vi "FlexMag - 24-03-2023.vi"() -> ()   [LabVIEW 2018] (continued)
              }
              frame True {
                w13696 = FALSE ("CH1_Trns_BP_Left_DO")
                w13698 = FALSE
                w13699 = FALSE
                w13697 = FALSE ("CH1_CC_DO")
                n8105 = local write "Buzzer DO"(TRUE ("Buzzer DO")) -> ()
                n8106 = local write "1-2 tr"(w13699) -> ()
                n8107 = local write "1-3 tr"(w13699) -> ()
                n8108 = local write "1-4 tr"(w13699) -> ()
                n8109 = local write "2-1 tr"(w13699) -> ()
                n8110 = local write "2-3 tr"(w13699) -> ()
                n8111 = local write "2-4 tr"(w13699) -> ()
                n8112 = local write "3-1 tr"(w13699) -> ()
                n8113 = local write "3-2 tr"(w13699) -> ()
                n8114 = local write "3-4 tr"(w13699) -> ()
                n8115 = local write "4-1 tr"(w13699) -> ()
                n8116 = local write "4-2 tr"(w13699) -> ()
                n8117 = local write "4-3 tr"(w13699) -> ()
                n8118 = local write "Casette_Servo_Start/Stop DO"(FALSE ("Casette_Servo_Start/Stop DO")) -> ()
                n8119 = local write "CH3_Trns_BP_Left_DO"(w13696) -> ()
                n8120 = local write "CH3_Trns_BP_Right_DO"(w13696) -> ()
                n8121 = local write "CH3_CC_DO"(w13697) -> ()
                n8122 = local write "ch3 pumpdown alg"(w13697) -> ()
                n8123 = local write "Pump Down CH3"(w13697) -> ()
                n8124 = local write "ch3 shutdown alg"(w13697) -> ()
                n8125 = local write "Shut Down CH3"(w13697) -> ()
                n8126 = local write "ch1-2 transfer"(w13698) -> ()
                n8127 = local write "ch2-3 transfer"(w13698) -> ()
                n8128 = local write "ch3-4 transfer"(w13698) -> ()
                n8129 = local write "ch2-1 transfer"(w13698) -> ()
                n8130 = local write "ch3-2 transfer"(w13698) -> ()
                n8131 = local write "ch4-3 transfer"(w13698) -> ()
              }
            }
            n8132 = case shown="True" w13676 {
              frame False {
              }
              frame True {
                w13692 = TRUE ("Buzzer DO")
                n8133 = local write "Tp3 auto stop"(w13692) -> ()
                n8134 = local write "pcgv3 auto close"(w13692) -> ()
                n8135 = local write "Dc_auto_off"(FALSE ("Dc_auto_off")) -> ()
                n8136 = local write "System Status"("CH3 ABORTED" ("System Status")) -> ()
              }
            }
            n8137 = case shown="True" w13669 {
              frame False {
              }
              frame True {
                n8138 = local write "CH3_PL_VBV_DO"(TRUE) -> ()
                n8139 = local write "CH3_MP_DO"(FALSE ("Buzzer DO")) -> ()
              }
            }
          }
        }
        n8140 = feedback-in #313(w13665) -> ()
      }
    }
  }
  n8141 = VISA Close(VISA resource name=w102, error in (no error)=w101) -> ()  [unwired: 1 out]
  n8142 = VISA Close(VISA resource name=w84, error in (no error)=w85) -> ()  [unwired: 1 out]
  n8143 = VISA Close(VISA resource name=w82, error in (no error)=w83) -> ()  [unwired: 1 out]
  n8144 = VISA Close(VISA resource name=w92, error in (no error)=w91) -> ()  [unwired: 1 out]
  n8145 = while {
    stop <- FALSE stop-if-true
    n8146 = Build Array(FALSE, "ch1-2 transfer", "ch2-3 transfer", "ch3-4 transfer", "ch2-1 transfer", "ch3-2 transfer", "ch4-3 transfer") -> (w13744:bool[])
    n8147 = Boolean Array To Number(Boolean array=w13744) -> (number=w13743:u32)
    n8148 = Wait Until Next ms Multiple(millisecond multiple=u32 300) -> ()  [unwired: 1 out]
    n8149 = Mantissa & Exponent(0:w13743) -> (2:w13742:dbl)  [unwired: 1 out]
    n8150 = case shown="1" w13742 {
      frame 0, Default {
      }
      frame 1 {
        n8151 = local read "ABORT"() -> (w13747:bool)
        n8152 = case shown="False" w13747 {
          frame False {
            n8153 = stacked-sequence {
              frame #0 {
                n8154 = local read "ch1-2 transfer"() -> (w13748:bool)
                n8155 = case shown="True" w13748 {
                  frame False {
                  }
                  frame True {
                    n8156 = local read "present location"() -> (w13751:dbl)
                    n8157 = Wait (ms)(milliseconds to wait=u32 100) -> ()  [unwired: 1 out]
                    n8158 = Equal?(x=w13751, y=1.0) -> (x = y?=w13752:bool)
                    n8159 = case shown="True" w13752 {
                      frame False {
                        n8160 = local write "trns error"(TRUE ("TRNS error")) -> ()
                        n8161 = local write "Warning Message"("Transfer process canceled!\nCassette is not in CH1 " ("Warning Message")) -> ()
                      }
                      frame True {
                        n8162 = local write "System Status"("CH1 to CH2  Transfer in Progress" ("System Status")) -> ()
                      }
                    }
                  }
                }
              }
              frame #1 {
                n8163 = local read "ch1-2 transfer"() -> (w13756:bool)
                n8164 = case shown="True" w13756 {
                  frame False {
                  }
                  frame True {
                    n8165 = stacked-sequence {
                      frame #0 {
                        n8166 = local read "ABORT"() -> (w13757:bool)
                        n8167 = case shown="False" w13757 {
                          frame False {
                            n8168 = local write "trns pre check"(TRUE ("trns pre check")) -> ()
                          }
                          frame True {
                          }
                        }
                      }
                      frame #1 {
                        n8169 = Wait (ms)(milliseconds to wait=u32 1000) -> ()  [unwired: 1 out]
                      }
                      frame #2 {
                        n8170 = while {
                          i -> [w13765]
                          stop <- w13762 stop-if-true
                          # "10 min"
                          n8171 = local read "trns pre check"() -> (w13769:bool)
                          n8172 = local read "ch1-2 transfer"() -> (w13761:bool)
                          n8173 = local read "ABORT"() -> (w13763:bool)
                          n8174 = Greater Or Equal?(x=w13765, y=u32 2000 ("millisecond multiple")) -> (x >= y?=w13764:bool)
                          n8175 = Not(x=w13769) -> (.not. x?=w13768:bool)
                          n8176 = Not(x=w13761) -> (.not. x?=w13760:bool)
                          n8177 = Compound Arithmetic op=OR(w13764, w13768, w13763, w13760) -> (w13762:bool)
                          n8178 = Wait Until Next ms Multiple(millisecond multiple=u32 300) -> ()  [unwired: 1 out]
                        }
                      }
                    }
                  }
                }
              }
              frame #2 {
                n8179 = local read "ch1-2 transfer"() -> (w13770:bool)
                n8180 = case shown="True" w13770 {
                  frame False {
                  }
                  frame True {
                    n8181 = local read "trns V?"() -> (w13771:bool)
                    n8182 = case shown="False" w13771 {
                      frame False {
                        n8183 = stacked-sequence {
                          frame #0 {
                            n8184 = local read "ABORT"() -> (w13772:bool)
                            n8185 = case shown="False" w13772 {
                              frame False {
                                w13774 = FALSE ("CH1_CH_ATM_DO")
                                n8186 = local write "CH1_CH_ATM_DO"(w13774) -> ()
                                n8187 = local write "CH2_CH_ATM_DO"(w13774) -> ()
                                n8188 = Wait (ms)(milliseconds to wait=u32 3000) -> ()  [unwired: 1 out]
                              }
                              frame True {
                              }
                            }
                          }
                          frame #1 {
                            n8189 = while {
                              i -> [w13777]
                              stop <- w13778 stop-if-true
                              n8190 = Greater Or Equal?(x=w13777, y=200) -> (x >= y?=w13775:bool)
                              n8191 = case shown="True" w13775 {
                                frame False {
                                }
                                frame True {
                                n8192 = local write "Warning Message"("Transfer process canceled!\nChambers should be on Atmosphere Pressure" ("Warning Message")) -> ()
                                n8193 = local write "trns error"(TRUE ("TRNS error")) -> ()
                                }
                              }
                              n8194 = local read "CH1_CH_ATM_DI"() -> (w13782:bool)
                              n8195 = local read "CH2_CH_ATM_DI"() -> (w13781:bool)
                              n8196 = local read "ch1-2 transfer"() -> (w13784:bool)
                              n8197 = local read "ABORT"() -> (w13785:bool)
                              n8198 = Not(x=w13784) -> (.not. x?=w13783:bool)
                              n8199 = And(x=w13782, y=w13781) -> (x .and. y?=w13780:bool)
                              n8200 = Compound Arithmetic op=OR(w13780, w13785, w13783) -> (w13778:bool)
                              n8201 = Wait Until Next ms Multiple(millisecond multiple=u32 300) -> ()  [unwired: 1 out]
                            }
                          }
                        }
                      }
                      frame True {
                        n8202 = local read "ch1 ch pg torr"() -> (w13794:dbl)
                        n8203 = local read "ch2 ch pg torr"() -> (w13791:dbl)
                        n8204 = Greater Or Equal?(x=w13794, y=0.5) -> (x >= y?=w13790:bool)
                        n8205 = Greater Or Equal?(x=w13791, y=0.5) -> (x >= y?=w13789:bool)
                        n8206 = Or(x=w13790, y=w13789) -> (x .or. y?=w13788:bool)
                        n8207 = local write "trns error"(w13788) -> ()
                      }
                    }
                  }
                }
              }
              frame #3 {
                n8208 = local read "ch1-2 transfer"() -> (w13795:bool)
                n8209 = case shown="True" w13795 {
                  frame False {
                  }
                  frame True {
                    n8210 = local read "ABORT"() -> (w13796:bool)
                    n8211 = case shown="False" w13796 {
                      frame False {
                        n8212 = while {
                          i -> [w13801]
                          stop <- w13802 stop-if-true
                          n8213 = Greater Or Equal?(x=w13801, y=100) -> (x >= y?=w13799:bool)
                          n8214 = case shown="True" w13799 {
                            frame False {
                            }
                            frame True {
                              n8215 = local write "trns error"(TRUE ("TRNS error")) -> ()
                              n8216 = local write "Warning Message"("Transfer process canceled!\nCH1 Trns BP Left couln't be opened" ("Warning Message")) -> ()
                            }
                          }
                          n8217 = local read "CH1_Trns_BP_Left_DI"() -> (w13798:bool)
                          n8218 = case shown="False" w13798 {
                            tunnel: [FALSE ("CH1_Trns_BP_Left_DO") TRUE ("CH1_Trns_BP_Left_DO")] -> w13797
                            frame False {
                              n8219 = Wait Until Next ms Multiple(millisecond multiple=u32 200) -> ()  [unwired: 1 out]
                              n8220 = local write "CH1_Trns_BP_Left_DO"(TRUE ("CH1_Trns_BP_Left_DO")) -> ()
                            }
                            frame True {
                            }
                          }
                          n8221 = local read "ch1-2 transfer"() -> (w13805:bool)
                          n8222 = local read "ABORT"() -> (w13804:bool)
                          n8223 = Not(x=w13805) -> (.not. x?=w13803:bool)
                          n8224 = Compound Arithmetic op=OR(w13797, w13804, w13803) -> (w13802:bool)
                        }
                      }
                      frame True {
                      }
                    }
                  }
                }
              }
              frame #4 {
                n8225 = local read "ch1-2 transfer"() -> (w13812:bool)
                n8226 = case shown="True" w13812 {
                  frame False {
                  }
                  frame True {
                    n8227 = local read "ABORT"() -> (w13813:bool)
                    n8228 = case shown="False" w13813 {
                      frame False {
                        n8229 = local write "trns 1-2 led 1"(TRUE ("trns 1-2 led 1")) -> ()
                        n8230 = Wait (ms)(milliseconds to wait=u32 100) -> ()  [unwired: 1 out]
                      }
                      frame True {
                      }
                    }
                  }
                }
              }
              frame #5 {
                n8231 = local read "ch1-2 transfer"() -> (w13816:bool)
                n8232 = case shown="True" w13816 {
                  frame False {
                  }
                  frame True {
                    n8233 = local read "ABORT"() -> (w13817:bool)
                    n8234 = case shown="False" w13817 {
                      frame False {
                        n8235 = while {
                          i -> [w13822]
                          stop <- w13823 stop-if-true
                          n8236 = Greater Or Equal?(x=w13822, y=100) -> (x >= y?=w13820:bool)
                          n8237 = case shown="True" w13820 {
                            frame False {
                            }
                            frame True {
                              n8238 = local write "trns error"(TRUE ("TRNS error")) -> ()
                              n8239 = local write "Warning Message"("Transfer process canceled!\nCH2 Trns BP Right couln't be opened" ("Warning Message")) -> ()
                            }
                          }
                          n8240 = local read "CH2_Trns_BP_Right_DI"() -> (w13819:bool)
                          n8241 = case shown="False" w13819 {
                            tunnel: [FALSE ("CH1_Trns_BP_Left_DO") TRUE ("CH1_Trns_BP_Left_DO")] -> w13818
                            frame False {
                              n8242 = Wait Until Next ms Multiple(millisecond multiple=u32 200) -> ()  [unwired: 1 out]
                              n8243 = local write "CH2_Trns_BP_Right_DO"(TRUE ("CH1_Trns_BP_Left_DO")) -> ()
                            }
                            frame True {
                            }
                          }
                          n8244 = local read "ch1-2 transfer"() -> (w13826:bool)
                          n8245 = local read "ABORT"() -> (w13825:bool)
                          n8246 = Not(x=w13826) -> (.not. x?=w13824:bool)
                          n8247 = Compound Arithmetic op=OR(w13818, w13825, w13824) -> (w13823:bool)
                        }
                      }
                      frame True {
                      }
                    }
                  }
                }
              }
              frame #6 {
                n8248 = local read "ch1-2 transfer"() -> (w13833:bool)
                n8249 = case shown="True" w13833 {
                  frame False {
                  }
                  frame True {
                    n8250 = local read "ABORT"() -> (w13834:bool)
                    n8251 = case shown="False" w13834 {
                      frame False {
                        n8252 = local write "trns 1-2 led 2"(TRUE ("trns 1-2 led 1")) -> ()
                        n8253 = Wait (ms)(milliseconds to wait=u32 100) -> ()  [unwired: 1 out]
                      }
                      frame True {
                      }
                    }
                  }
                }
              }
              frame #7 {
                n8254 = local read "ch1-2 transfer"() -> (w13837:bool)
                n8255 = case shown="True" w13837 {
                  frame False {
                  }
                  frame True {
                    n8256 = local read "ABORT"() -> (w13838:bool)
                    n8257 = case shown="False" w13838 {
                      frame False {
                        n8258 = stacked-sequence {
                          frame #0 {
                            n8259 = local write "CH1_Trns_Gv_Close_DO"(FALSE ("CH1_Trns_Gv_Close_DO")) -> ()
                            n8260 = Wait (ms)(milliseconds to wait=u32 100) -> ()  [unwired: 1 out]
                          }
                          frame #1 {
                            n8261 = while {
                              i -> [w13845]
                              stop <- w13846 stop-if-true
                              n8262 = Greater Or Equal?(x=w13845, y=600) -> (x >= y?=w13843:bool)
                              n8263 = case shown="True" w13843 {
                                frame False {
                                }
                                frame True {
                                n8264 = local write "trns error"(TRUE ("TRNS error")) -> ()
                                n8265 = local write "Warning Message"("Transfer process canceled!\nCH1-CH2 Trns GV couln't be opened" ("Warning Message")) -> ()
                                }
                              }
                              n8266 = local read "CH1_Trns_Gv_Open_DI"() -> (w13842:bool)
                              n8267 = case shown="False" w13842 {
                                tunnel: [FALSE ("CH1_Trns_BP_Left_DO") TRUE ("CH1_Trns_BP_Left_DO")] -> w13841
                                frame False {
                                n8268 = local write "CH1_Trns_Gv_Open_DO"(TRUE ("CH1_Trns_BP_Left_DO")) -> ()
                                n8269 = Wait Until Next ms Multiple(millisecond multiple=u32 200) -> ()  [unwired: 1 out]
                                }
                                frame True {
                                }
                              }
                              n8270 = local read "ch1-2 transfer"() -> (w13849:bool)
                              n8271 = local read "ABORT"() -> (w13848:bool)
                              n8272 = Not(x=w13849) -> (.not. x?=w13847:bool)
                              n8273 = Compound Arithmetic op=OR(w13841, w13848, w13847) -> (w13846:bool)
                            }
                          }
                        }
                      }
                      frame True {
                      }
                    }
                  }
                }
              }
              frame #8 {
                n8274 = local read "ch1-2 transfer"() -> (w13856:bool)
                n8275 = case shown="True" w13856 {
                  frame False {
                  }
                  frame True {
                    n8276 = local read "ABORT"() -> (w13857:bool)
                    n8277 = case shown="False" w13857 {
                      frame False {
                        n8278 = local write "trns 1-2 led 3"(TRUE ("trns 1-2 led 1")) -> ()
                        n8279 = Wait (ms)(milliseconds to wait=u32 100) -> ()  [unwired: 1 out]
                      }
                      frame True {
                      }
                    }
                  }
                }
              }
              frame #9 {
                n8280 = local read "ch1-2 transfer"() -> (w13860:bool)
                n8281 = case shown="True" w13860 {
                  frame False {
                  }
                  frame True {
                    n8282 = local read "ABORT"() -> (w13861:bool)
                    n8283 = case shown="False" w13861 {
                      frame False {
                        n8284 = while {
                          i -> [w13866]
                          stop <- w13867 stop-if-true
                          n8285 = Greater Or Equal?(x=w13866, y=100) -> (x >= y?=w13864:bool)
                          n8286 = case shown="True" w13864 {
                            frame False {
                            }
                            frame True {
                              n8287 = local write "trns error"(TRUE ("TRNS error")) -> ()
                              n8288 = local write "Warning Message"("Transfer process canceled!\nCH1 TGV Control Problem" ("Warning Message")) -> ()
                            }
                          }
                          n8289 = local read "CH1_TGV_Control_DI"() -> (w13863:bool)
                          n8290 = case shown="True" w13863 {
                            tunnel: [TRUE ("CH1_Trns_BP_Left_DO") FALSE ("CH1_Trns_BP_Left_DO")] -> w13862
                            frame False {
                            }
                            frame True {
                              n8291 = Wait Until Next ms Multiple(millisecond multiple=u32 200) -> ()  [unwired: 1 out]
                              n8292 = local write "CH1_TGV_Control_DO"(FALSE ("CH1_Trns_BP_Left_DO")) -> ()
                            }
                          }
                          n8293 = local read "ch1-2 transfer"() -> (w13870:bool)
                          n8294 = local read "ABORT"() -> (w13869:bool)
                          n8295 = Not(x=w13870) -> (.not. x?=w13868:bool)
                          n8296 = Compound Arithmetic op=OR(w13862, w13869, w13868) -> (w13867:bool)
                        }
                      }
                      frame True {
                      }
                    }
                  }
                }
              }
              frame #10 {
                n8297 = local read "ch1-2 transfer"() -> (w13877:bool)
                n8298 = case shown="True" w13877 {
                  frame False {
                  }
                  frame True {
                    n8299 = local read "ABORT"() -> (w13878:bool)
                    n8300 = case shown="False" w13878 {
                      frame False {
                        n8301 = local write "trns 1-2 led 4"(TRUE ("trns 1-2 led 1")) -> ()
                        n8302 = Wait (ms)(milliseconds to wait=u32 100) -> ()  [unwired: 1 out]
                      }
                      frame True {
                      }
                    }
                  }
                }
              }
              frame #11 {
                n8303 = local read "ch1-2 transfer"() -> (w13881:bool)
                n8304 = case shown="True" w13881 {
                  frame False {
                  }
                  frame True {
                    n8305 = local read "ABORT"() -> (w13882:bool)
                    n8306 = case shown="False" w13882 {
                      frame False {
                        n8307 = while {
                          i -> [w13887]
                          stop <- w13888 stop-if-true
                          n8308 = local read "CH2_Trns_Interlock_DI"() -> (w13883:bool)
                          n8309 = Greater Or Equal?(x=w13887, y=100) -> (x >= y?=w13885:bool)
                          n8310 = case shown="True" w13885 {
                            frame False {
                            }
                            frame True {
                              n8311 = local write "Warning Message"("Transfer process canceled!\nCH2 Interlock problem" ("Warning Message")) -> ()
                              n8312 = local write "trns error"(TRUE ("TRNS error")) -> ()
                            }
                          }
                          n8313 = case shown="False" w13883 {
                            tunnel: [w13892 TRUE ("CH1_Trns_BP_Left_DO")] -> w13884
                            frame False {
                              n8314 = local read "CH2_TGV_Control_DI"() -> (w13893:bool)
                              n8315 = case shown="False" w13893 {
                                tunnel: [FALSE ("CH1_Trns_BP_Left_DO") TRUE ("CH1_Trns_BP_Left_DO")] -> w13892
                                frame False {
                                n8316 = Wait Until Next ms Multiple(millisecond multiple=u32 200) -> ()  [unwired: 1 out]
                                n8317 = local write "CH2_TGV_Control_DO"(TRUE ("CH1_Trns_BP_Left_DO")) -> ()
                                }
                                frame True {
                                }
                              }
                            }
                            frame True {
                            }
                          }
                          n8318 = local read "ch1-2 transfer"() -> (w13891:bool)
                          n8319 = local read "ABORT"() -> (w13890:bool)
                          n8320 = Not(x=w13891) -> (.not. x?=w13889:bool)
                          n8321 = Compound Arithmetic op=OR(w13884, w13890, w13889) -> (w13888:bool)
                        }
                      }
                      frame True {
                      }
                    }
                  }
                }
              }
              frame #12 {
                n8322 = local read "ch1-2 transfer"() -> (w13901:bool)
                n8323 = case shown="True" w13901 {
                  frame False {
                  }
                  frame True {
                    n8324 = local read "ABORT"() -> (w13902:bool)
                    n8325 = case shown="False" w13902 {
                      frame False {
                        w13903 = TRUE ("CH1_Right_Limit_DO")
                        n8326 = local write "trns 1-2 led 5"(TRUE ("trns 1-2 led 1")) -> ()
                        n8327 = Wait (ms)(milliseconds to wait=u32 100) -> ()  [unwired: 1 out]
                        n8328 = local write "CH1_Right_Limit_DO"(w13903) -> ()
                        n8329 = local write "CH1_Right_Slow_DO"(w13903) -> ()
                      }
                      frame True {
                      }
                    }
                  }
                }
              }
              frame #13 {
                n8330 = local read "ch1-2 transfer"() -> (w13906:bool)
                n8331 = case shown="True" w13906 {
                  frame False {
                  }
                  frame True {
                    n8332 = local read "ABORT"() -> (w13907:bool)
                    n8333 = case shown="False" w13907 {
                      frame False {
                        n8334 = while {
                          i -> [w13912]
                          stop <- w13913 stop-if-true
                          n8335 = local read "CH3_Trns_Interlock_DI"() -> (w13908:bool)
                          n8336 = Greater Or Equal?(x=w13912, y=100) -> (x >= y?=w13910:bool)
                          n8337 = case shown="True" w13910 {
                            frame False {
                            }
                            frame True {
                              n8338 = local write "Warning Message"("Transfer process canceled!\nCH3 Interlock problem" ("Warning Message")) -> ()
                              n8339 = local write "trns error"(TRUE ("TRNS error")) -> ()
                            }
                          }
                          n8340 = case shown="False" w13908 {
                            tunnel: [w13917 TRUE ("CH1_Trns_BP_Left_DO")] -> w13909
                            frame False {
                              n8341 = local read "CH3_TGV_Control_DI"() -> (w13918:bool)
                              n8342 = case shown="False" w13918 {
                                tunnel: [FALSE ("CH1_Trns_BP_Left_DO") TRUE ("CH1_Trns_BP_Left_DO")] -> w13917
                                frame False {
                                n8343 = Wait Until Next ms Multiple(millisecond multiple=u32 200) -> ()  [unwired: 1 out]
                                n8344 = local write "CH3_TGV_Control_DO"(TRUE ("CH1_Trns_BP_Left_DO")) -> ()
                                }
                                frame True {
                                }
                              }
                            }
                            frame True {
                            }
                          }
                          n8345 = local read "ch1-2 transfer"() -> (w13916:bool)
                          n8346 = local read "ABORT"() -> (w13915:bool)
                          n8347 = Not(x=w13916) -> (.not. x?=w13914:bool)
                          n8348 = Compound Arithmetic op=OR(w13909, w13915, w13914) -> (w13913:bool)
                        }
                      }
                      frame True {
                      }
                    }
                  }
                }
              }
              frame #14 {
                n8349 = local read "ch1-2 transfer"() -> (w13926:bool)
                n8350 = case shown="True" w13926 {
                  frame False {
                  }
                  frame True {
                    n8351 = local read "ABORT"() -> (w13927:bool)
                    n8352 = case shown="False" w13927 {
                      frame False {
                        n8353 = local write "trns 1-2 led 6"(TRUE ("trns 1-2 led 1")) -> ()
                        n8354 = Wait (ms)(milliseconds to wait=u32 100) -> ()  [unwired: 1 out]
                      }
                      frame True {
                      }
                    }
                  }
                }
              }
              frame #15 {
                n8355 = local read "ch1-2 transfer"() -> (w13930:bool)
                n8356 = case shown="True" w13930 {
                  frame False {
                  }
                  frame True {
                    n8357 = local read "ABORT"() -> (w13931:bool)
                    n8358 = case shown="False" w13931 {
                      frame False {
                        n8359 = while {
                          i -> [w13936]
                          stop <- w13937 stop-if-true
                          n8360 = local read "CH4_Trns_Interlock_DI"() -> (w13932:bool)
                          n8361 = Greater Or Equal?(x=w13936, y=100) -> (x >= y?=w13934:bool)
                          n8362 = case shown="True" w13934 {
                            frame False {
                            }
                            frame True {
                              n8363 = local write "Warning Message"("Transfer process canceled!\nCH4 Interlock problem" ("Warning Message")) -> ()
                              n8364 = local write "trns error"(TRUE ("TRNS error")) -> ()
                            }
                          }
                          n8365 = case shown="False" w13932 {
                            tunnel: [w13941 TRUE ("CH1_Trns_BP_Left_DO")] -> w13933
                            frame False {
                              n8366 = local read "CH4_TGV_Control_DI"() -> (w13942:bool)
                              n8367 = case shown="False" w13942 {
                                tunnel: [FALSE ("CH1_Trns_BP_Left_DO") TRUE ("CH1_Trns_BP_Left_DO")] -> w13941
                                frame False {
                                n8368 = Wait Until Next ms Multiple(millisecond multiple=u32 200) -> ()  [unwired: 1 out]
                                n8369 = local write "CH4_TGV_Control_DO"(TRUE ("CH1_Trns_BP_Left_DO")) -> ()
                                }
                                frame True {
                                }
                              }
                            }
                            frame True {
                            }
                          }
                          n8370 = local read "ch1-2 transfer"() -> (w13940:bool)
                          n8371 = local read "ABORT"() -> (w13939:bool)
                          n8372 = Not(x=w13940) -> (.not. x?=w13938:bool)
                          n8373 = Compound Arithmetic op=OR(w13933, w13939, w13938) -> (w13937:bool)
                        }
                      }
                      frame True {
                      }
                    }
                  }
                }
              }
              frame #16 {
                n8374 = local read "ch1-2 transfer"() -> (w13950:bool)
                n8375 = case shown="True" w13950 {
                  frame False {
                  }
                  frame True {
                    n8376 = local read "ABORT"() -> (w13951:bool)
                    n8377 = case shown="False" w13951 {
                      frame False {
                        n8378 = local write "trns 1-2 led 7"(TRUE ("trns 1-2 led 1")) -> ()
                        n8379 = Wait (ms)(milliseconds to wait=u32 100) -> ()  [unwired: 1 out]
                      }
                      frame True {
                      }
                    }
                  }
                }
              }
              frame #17 {
                n8380 = local read "ch1-2 transfer"() -> (w13954:bool)
                n8381 = case shown="True" w13954 {
                  frame False {
                  }
                  frame True {
                    n8382 = local read "ABORT"() -> (w13955:bool)
                    n8383 = case shown="False" w13955 {
                      frame False {
                        n8384 = while {
                          i -> [w13959]
                          stop <- w13960 stop-if-true
                          n8385 = Greater Or Equal?(x=w13959, y=100) -> (x >= y?=w13957:bool)
                          n8386 = disable-structure shown="Enabled" {
                            disable-tunnel: [w13965 w13970] -> w13956
                            frame Disabled {
                              n8387 = local read "Cnt_Right_Slow DI"() -> (w13964:bool)
                              n8388 = case shown="False" w13964 {
                                tunnel: [FALSE ("CH1_Trns_BP_Left_DO") TRUE ("CH1_Trns_BP_Left_DO")] -> w13965
                                frame False {
                                n8389 = Wait Until Next ms Multiple(millisecond multiple=u32 200) -> ()  [unwired: 1 out]
                                n8390 = local write "Cnt_Right_Slow DO"(TRUE ("CH1_Trns_BP_Left_DO")) -> ()
                                }
                                frame True {
                                }
                              }
                            }
                            frame Enabled {
                              n8391 = local read "CH1_Right_Limit_DI"() -> (w13971:bool)
                              n8392 = case shown="True" w13971 {
                                tunnel: [TRUE FALSE ("CH1_Right_Limit_DO")] -> w13970
                                frame False {
                                }
                                frame True {
                                n8393 = Wait Until Next ms Multiple(millisecond multiple=u32 200) -> ()  [unwired: 1 out]
                                n8394 = local write "CH1_Right_Limit_DO"(TRUE ("CH1_Right_Limit_DO")) -> ()
                                }
                              }
                            }
                          }
                          n8395 = case shown="True" w13957 {
                            frame False {
                            }
                            frame True {
                              n8396 = local write "Warning Message"("Transfer process canceled!\nRight Slow Sensor problem" ("Warning Message")) -> ()
                              n8397 = local write "trns error"(TRUE ("TRNS error")) -> ()
                            }
                          }
                          n8398 = local read "ch1-2 transfer"() -> (w13963:bool)
                          n8399 = local read "ABORT"() -> (w13962:bool)
                          n8400 = Not(x=w13963) -> (.not. x?=w13961:bool)
                          n8401 = Compound Arithmetic op=OR(w13956, w13962, w13961) -> (w13960:bool)
                        }
                      }
                      frame True {
                      }
                    }
                  }
                }
              }
              frame #18 {
                n8402 = local read "ch1-2 transfer"() -> (w13978:bool)
                n8403 = case shown="True" w13978 {
                  frame False {
                  }
                  frame True {
                    n8404 = local read "ABORT"() -> (w13979:bool)
                    n8405 = case shown="False" w13979 {
                      frame False {
                        n8406 = local write "trns 1-2 led 8"(TRUE ("trns 1-2 led 1")) -> ()
                        n8407 = Wait (ms)(milliseconds to wait=u32 100) -> ()  [unwired: 1 out]
                      }
                      frame True {
                      }
                    }
                  }
                }
              }
              frame #19 {
                n8408 = local read "ch1-2 transfer"() -> (w13982:bool)
                n8409 = case shown="True" w13982 {
                  frame False {
                  }
                  frame True {
                    n8410 = local read "ABORT"() -> (w13983:bool)
                    n8411 = case shown="False" w13983 {
                      frame False {
                        n8412 = while {
                          i -> [w13987]
                          stop <- w13988 stop-if-true
                          n8413 = Greater Or Equal?(x=w13987, y=100) -> (x >= y?=w13985:bool)
                          n8414 = case shown="True" w13985 {
                            frame False {
                            }
                            frame True {
                              n8415 = local write "Warning Message"("Transfer process canceled!\nRight Limit Sensor problem" ("Warning Message")) -> ()
                              n8416 = local write "trns error"(TRUE ("TRNS error")) -> ()
                            }
                          }
                          n8417 = disable-structure shown="Enabled" {
                            disable-tunnel: [w13993 w13998] -> w13984
                            frame Disabled {
                              n8418 = local read "Cnt_Right_Limit DI"() -> (w13992:bool)
                              n8419 = case shown="False" w13992 {
                                tunnel: [FALSE ("CH1_Trns_BP_Left_DO") TRUE ("CH1_Trns_BP_Left_DO")] -> w13993
                                frame False {
                                n8420 = Wait Until Next ms Multiple(millisecond multiple=u32 200) -> ()  [unwired: 1 out]
                                n8421 = local write "Cnt_Right_Limit DO"(TRUE ("CH1_Trns_BP_Left_DO")) -> ()
                                }
                                frame True {
                                }
                              }
                            }
                            frame Enabled {
                              n8422 = local read "CH1_Right_Slow_DI"() -> (w13999:bool)
                              n8423 = case shown="True" w13999 {
                                tunnel: [TRUE FALSE ("CH1_Right_Slow_DO")] -> w13998
                                frame False {
                                }
                                frame True {
                                n8424 = Wait Until Next ms Multiple(millisecond multiple=u32 200) -> ()  [unwired: 1 out]
                                n8425 = local write "CH1_Right_Slow_DO"(TRUE ("CH1_Right_Slow_DO")) -> ()
                                }
                              }
                            }
                          }
                          n8426 = local read "ch1-2 transfer"() -> (w13991:bool)
                          n8427 = local read "ABORT"() -> (w13990:bool)
                          n8428 = Not(x=w13991) -> (.not. x?=w13989:bool)
                          n8429 = Compound Arithmetic op=OR(w13984, w13990, w13989) -> (w13988:bool)
                        }
                      }
                      frame True {
                      }
                    }
                  }
                }
              }
              frame #20 {
                n8430 = local read "ch1-2 transfer"() -> (w14006:bool)
                n8431 = case shown="True" w14006 {
                  frame False {
                  }
                  frame True {
                    n8432 = local read "ABORT"() -> (w14007:bool)
                    n8433 = case shown="False" w14007 {
                      frame False {
                        n8434 = local write "trns 1-2 led 9"(TRUE ("trns 1-2 led 1")) -> ()
                        n8435 = Wait (ms)(milliseconds to wait=u32 100) -> ()  [unwired: 1 out]
                      }
                      frame True {
                      }
                    }
                  }
                }
              }
              frame #21 {
                n8436 = local read "ch1-2 transfer"() -> (w14010:bool)
                n8437 = case shown="True" w14010 {
                  frame False {
                  }
                  frame True {
                    n8438 = local read "ABORT"() -> (w14011:bool)
                    n8439 = case shown="False" w14011 {
                      frame False {
                        n8440 = disable-structure shown="Enabled" {
                          frame Disabled {
                            n8441 = while {
                              i -> [w14016]
                              stop <- w14017 stop-if-true
                              n8442 = Greater Or Equal?(x=w14016, y=100) -> (x >= y?=w14014:bool)
                              n8443 = case shown="True" w14014 {
                                frame False {
                                }
                                frame True {
                                n8444 = local write "Warning Message"("Transfer process canceled!\nLeft Slow Sensor problem" ("Warning Message")) -> ()
                                n8445 = local write "trns error"(TRUE ("TRNS error")) -> ()
                                }
                              }
                              n8446 = local read "Cnt_Left_Slow DI"() -> (w14012:bool)
                              n8447 = case shown="True" w14012 {
                                tunnel: [TRUE ("CH1_Trns_BP_Left_DO") FALSE ("CH1_Trns_BP_Left_DO")] -> w14013
                                frame False {
                                }
                                frame True {
                                n8448 = Wait Until Next ms Multiple(millisecond multiple=u32 200) -> ()  [unwired: 1 out]
                                n8449 = local write "Cnt_Left_Slow DO"(FALSE ("CH1_Trns_BP_Left_DO")) -> ()
                                }
                              }
                              n8450 = local read "ch1-2 transfer"() -> (w14020:bool)
                              n8451 = local read "ABORT"() -> (w14019:bool)
                              n8452 = Not(x=w14020) -> (.not. x?=w14018:bool)
                              n8453 = Compound Arithmetic op=OR(w14013, w14019, w14018) -> (w14017:bool)
                            }
                          }
                          frame Enabled {
                            w14028 = FALSE ("CH2_Right_Limit_DO")
                            w14029 = TRUE ("CH2_Right_Limit_DO")
                            n8454 = local write "CH2_Right_Limit_DO"(w14029) -> ()
                            n8455 = local write "CH2_Right_Slow_DO"(w14029) -> ()
                            n8456 = local write "CH2_Left_Slow_DO"(w14028) -> ()
                            n8457 = local write "CH2_Left_Limit_DO"(w14028) -> ()
                            n8458 = Wait (ms)(milliseconds to wait=u32 2000) -> ()  [unwired: 1 out]
                          }
                        }
                      }
                      frame True {
                      }
                    }
                  }
                }
              }
              frame #22 {
                n8459 = local read "ch1-2 transfer"() -> (w14030:bool)
                n8460 = case shown="True" w14030 {
                  frame False {
                  }
                  frame True {
                    n8461 = local read "ABORT"() -> (w14031:bool)
                    n8462 = case shown="False" w14031 {
                      frame False {
                        n8463 = local write "trns 1-2 led 10"(TRUE ("trns 1-2 led 1")) -> ()
                        n8464 = Wait (ms)(milliseconds to wait=u32 100) -> ()  [unwired: 1 out]
                      }
                      frame True {
                      }
                    }
                  }
                }
              }
              frame #23 {
                n8465 = local read "ch1-2 transfer"() -> (w14034:bool)
                n8466 = case shown="True" w14034 {
                  frame False {
                  }
                  frame True {
                    n8467 = local read "ABORT"() -> (w14035:bool)
                    n8468 = case shown="False" w14035 {
                      frame False {
                        n8469 = disable-structure shown="Disabled" {
                          frame Disabled {
                            n8470 = while {
                              i -> [w14040]
                              stop <- w14041 stop-if-true
                              n8471 = Greater Or Equal?(x=w14040, y=100) -> (x >= y?=w14038:bool)
                              n8472 = case shown="True" w14038 {
                                frame False {
                                }
                                frame True {
                                n8473 = local write "Warning Message"("Transfer process canceled!\nLeft Limit Sensor problem" ("Warning Message")) -> ()
                                n8474 = local write "trns error"(TRUE ("TRNS error")) -> ()
                                }
                              }
                              n8475 = local read "Cnt_Left_Limit DI"() -> (w14036:bool)
                              n8476 = case shown="True" w14036 {
                                tunnel: [TRUE ("CH1_Trns_BP_Left_DO") FALSE ("CH1_Trns_BP_Left_DO")] -> w14037
                                frame False {
                                }
                                frame True {
                                n8477 = Wait Until Next ms Multiple(millisecond multiple=u32 200) -> ()  [unwired: 1 out]
                                n8478 = local write "Cnt_Left_Limit DO"(FALSE ("CH1_Trns_BP_Left_DO")) -> ()
                                }
                              }
                              n8479 = local read "ch1-2 transfer"() -> (w14044:bool)
                              n8480 = local read "ABORT"() -> (w14043:bool)
                              n8481 = Not(x=w14044) -> (.not. x?=w14042:bool)
                              n8482 = Compound Arithmetic op=OR(w14037, w14043, w14042) -> (w14041:bool)
                            }
                          }
                          frame Enabled {
                          }
                        }
                      }
                      frame True {
                      }
                    }
                  }
                }
              }
              frame #24 {
                n8483 = local read "ch1-2 transfer"() -> (w14051:bool)
                n8484 = case shown="True" w14051 {
                  frame False {
                  }
                  frame True {
                    n8485 = local read "ABORT"() -> (w14052:bool)
                    n8486 = case shown="False" w14052 {
                      frame False {
                        n8487 = local write "trns 1-2 led 11"(TRUE ("trns 1-2 led 1")) -> ()
                        n8488 = Wait (ms)(milliseconds to wait=u32 100) -> ()  [unwired: 1 out]
                      }
                      frame True {
                      }
                    }
                  }
                }
              }
              frame #25 {
                n8489 = local read "ch1-2 transfer"() -> (w14055:bool)
                n8490 = case shown="True" w14055 {
                  frame False {
                  }
                  frame True {
                    n8491 = local read "ABORT"() -> (w14056:bool)
                    n8492 = case shown="False" w14056 {
                      frame False {
                        n8493 = while {
                          i -> [w14061]
                          stop <- w14062 stop-if-true
                          n8494 = Greater Or Equal?(x=w14061, y=100) -> (x >= y?=w14059:bool)
                          n8495 = case shown="True" w14059 {
                            frame False {
                            }
                            frame True {
                              n8496 = local write "Warning Message"("Transfer process canceled!\nCassette Servo Direction problem" ("Warning Message")) -> ()
                              n8497 = local write "trns error"(TRUE ("TRNS error")) -> ()
                            }
                          }
                          n8498 = local read "Casette_Servo_Left_Direction DI"() -> (w14057:bool)
                          n8499 = case shown="False" w14057 {
                            tunnel: [FALSE ("CH1_Trns_BP_Left_DO") TRUE ("CH1_Trns_BP_Left_DO")] -> w14058
                            frame False {
                              n8500 = local write "Casette_Servo_Left_Direction DO"(TRUE ("CH1_Trns_BP_Left_DO")) -> ()
                              n8501 = Wait Until Next ms Multiple(millisecond multiple=u32 200) -> ()  [unwired: 1 out]
                            }
                            frame True {
                            }
                          }
                          n8502 = local read "ch1-2 transfer"() -> (w14065:bool)
                          n8503 = local read "ABORT"() -> (w14064:bool)
                          n8504 = Not(x=w14065) -> (.not. x?=w14063:bool)
                          n8505 = Compound Arithmetic op=OR(w14058, w14064, w14063) -> (w14062:bool)
                        }
                      }
                      frame True {
                      }
                    }
                  }
                }
              }
              frame #26 {
                n8506 = local read "ch1-2 transfer"() -> (w14072:bool)
                n8507 = case shown="True" w14072 {
                  frame False {
                  }
                  frame True {
                    n8508 = local read "ABORT"() -> (w14073:bool)
                    n8509 = case shown="False" w14073 {
                      frame False {
                        n8510 = local write "trns 1-2 led 12"(TRUE ("trns 1-2 led 1")) -> ()
                        n8511 = Wait (ms)(milliseconds to wait=u32 100) -> ()  [unwired: 1 out]
                      }
                      frame True {
                      }
                    }
                  }
                }
              }
              frame #27 {
                n8512 = local read "ch1-2 transfer"() -> (w14076:bool)
                n8513 = case shown="True" w14076 {
                  frame False {
                  }
                  frame True {
                    n8514 = local read "ABORT"() -> (w14077:bool)
                    n8515 = case shown="False" w14077 {
                      frame False {
                        n8516 = stacked-sequence {
                          frame #0 {
                            n8517 = local read "Cst_Speed_High"() -> (w14078:dbl)
                            n8518 = Wait (ms)(milliseconds to wait=u32 100) -> ()  [unwired: 1 out]
                            n8519 = local write "Cassette_Servo_Speed AO"(w14078) -> ()
                          }
                          frame #1 {
                            n8520 = Wait (ms)(milliseconds to wait=u32 200) -> ()  [unwired: 1 out]
                          }
                          frame #2 {
                            n8521 = local write "Cassette_Servo_Speed Set"(TRUE ("Cassette_Servo_Speed Set")) -> ()
                          }
                          frame #3 {
                            n8522 = Wait (ms)(milliseconds to wait=u32 300) -> ()  [unwired: 1 out]
                          }
                        }
                      }
                      frame True {
                      }
                    }
                  }
                }
              }
              frame #28 {
                n8523 = local read "ch1-2 transfer"() -> (w14083:bool)
                n8524 = case shown="True" w14083 {
                  frame False {
                  }
                  frame True {
                    n8525 = local read "ABORT"() -> (w14084:bool)
                    n8526 = case shown="False" w14084 {
                      frame False {
                        n8527 = local write "trns 1-2 led 13"(TRUE ("trns 1-2 led 1")) -> ()
                        n8528 = Wait (ms)(milliseconds to wait=u32 100) -> ()  [unwired: 1 out]
                      }
                      frame True {
                      }
                    }
                  }
                }
              }
              frame #29 {
                n8529 = local read "ch1-2 transfer"() -> (w14087:bool)
                n8530 = case shown="True" w14087 {
                  frame False {
                  }
                  frame True {
                    n8531 = local read "ABORT"() -> (w14088:bool)
                    n8532 = case shown="False" w14088 {
                      frame False {
                        n8533 = while {
                          i -> [w14093]
                          stop <- w14094 stop-if-true
                          n8534 = Greater Or Equal?(x=w14093, y=100) -> (x >= y?=w14091:bool)
                          n8535 = case shown="True" w14091 {
                            frame False {
                            }
                            frame True {
                              n8536 = local write "Warning Message"("Transfer process canceled!\nCassette Servo Start problem" ("Warning Message")) -> ()
                              n8537 = local write "trns error"(TRUE ("TRNS error")) -> ()
                            }
                          }
                          n8538 = local read "Casette_Servo_Start/Stop DI"() -> (w14089:bool)
                          n8539 = case shown="False" w14089 {
                            tunnel: [FALSE ("CH1_Trns_BP_Left_DO") TRUE ("CH1_Trns_BP_Left_DO")] -> w14090
                            frame False {
                              n8540 = local write "Casette_Servo_Start/Stop DO"(TRUE ("CH1_Trns_BP_Left_DO")) -> ()
                              n8541 = Wait Until Next ms Multiple(millisecond multiple=u32 200) -> ()  [unwired: 1 out]
                            }
                            frame True {
                            }
                          }
                          n8542 = local read "ch1-2 transfer"() -> (w14097:bool)
                          n8543 = local read "ABORT"() -> (w14096:bool)
                          n8544 = Not(x=w14097) -> (.not. x?=w14095:bool)
                          n8545 = Compound Arithmetic op=OR(w14090, w14096, w14095) -> (w14094:bool)
                        }
                      }
                      frame True {
                      }
                    }
                  }
                }
              }
              frame #30 {
                n8546 = local read "ch1-2 transfer"() -> (w14104:bool)
                n8547 = case shown="True" w14104 {
                  frame False {
                  }
                  frame True {
                    n8548 = local read "ABORT"() -> (w14105:bool)
                    n8549 = case shown="False" w14105 {
                      frame False {
                        n8550 = local write "trns 1-2 led 14"(TRUE ("trns 1-2 led 1")) -> ()
                        n8551 = Wait (ms)(milliseconds to wait=u32 100) -> ()  [unwired: 1 out]
                      }
                      frame True {
                      }
                    }
                  }
                }
              }
              frame #31 {
                n8552 = local read "ch1-2 transfer"() -> (w14108:bool)
                n8553 = case shown="True" w14108 {
                  frame False {
                  }
                  frame True {
                    n8554 = local read "ABORT"() -> (w14109:bool)
                    n8555 = case shown="False" w14109 {
                      frame False {